vi "SaccadeAnalyser - Main.vi"(8 "error in (no error)":errorcluster, 11 "Data IN":T3={"Impulse Positions"=[{"Start"=5471, "End"=5813, "Impulse Plane"=enum."Yaw", "Impulse Direction +ve?"=FALSE, "Time offset"=0, "Amplitude offset"=0.0}, {"Start"=6974, "End"=7325, "Impulse Plane"=enum."Yaw", "Impulse Direction +ve?"=TRUE, "Time offset"=0, "Amplitude offset"=0.0}, {"Start"=7641, "End"=7980, "Impulse Plane"=enum."Yaw", "Impulse Direction +ve?"=FALSE, "Time offset"=0, "Amplitude offset"=0.0}, {"Start"=9060, "End"=9400, "Impulse Plane"=enum."Yaw", "Impulse Direction +ve?"=FALSE, "Time offset"=0, "Amplitude offset"=0.0}, {"Start"=9938, "End"=10282, "Impulse Plane"=enum."Yaw", "Impulse Direction +ve?"=FALSE, "Time offset"=0, "Amplitude offset"=0.0}, {"Start"=10800, "End"=11142, "Impulse Plane"=enum."Yaw", "Impulse Direction +ve?"=FALSE, "Time offset"=0, "Amplitude offset"=0.0}, {"Start"=11602, "End"=11942, "Impulse Plane"=enum."Yaw", "Impulse Direction +ve?"=TRUE, "Time offset"=0, "Amplitude offset"=0.0}, {"Start"=12449, "End"=12790, "Impulse Plane"=enum."Yaw", "Impulse Direction +ve?"=TRUE, "Time offset"=0, "Amplitude offset"=0.0}, {"Start"=13310, "End"=13653, "Impulse Plane"=enum."Yaw", "Impulse Direction +ve?"=TRUE, "Time offset"=0, "Amplitude offset"=0.0}, {"Start"=14191, "End"=14535, "Impulse Plane"=enum."Yaw", "Impulse Direction +ve?"=TRUE, "Time offset"=0, "Amplitude offset"=0.0}, {"Start"=15040, "End"=15380, "Impulse Plane"=enum."Yaw", "Impulse Direction +ve?"=FALSE, "Time offset"=0, "Amplitude offset"=0.0}, {"Start"=16780, "End"=17124, "Impulse Plane"=enum."Yaw", "Impulse Direction +ve?"=TRUE, "Time offset"=0, "Amplitude offset"=0.0}, {"Start"=17572, "End"=17913, "Impulse Plane"=enum."Yaw", "Impulse Direction +ve?"=FALSE, "Time offset"=0, "Amplitude offset"=0.0}, {"Start"=18369, "End"=18713, "Impulse Plane"=enum."Yaw", "Impulse Direction +ve?"=FALSE, "Time offset"=0, "Amplitude offset"=0.0}, {"Start"=19174, "End"=19519, "Impulse Plane"=enum."Yaw", "Impulse Direction +ve?"=FALSE, "Time offset"=0, "Amplitude offset"=0.0}, {"Start"=19928, "End"=20270, "Impulse Plane"=enum."Yaw", "Impulse Direction +ve?"=TRUE, "Time offset"=0, "Amplitude offset"=0.0}, {"Start"=20762, "End"=21121, "Impulse Plane"=enum."Yaw", "Impulse Direction +ve?"=FALSE, "Time offset"=0, "Amplitude offset"=0.0}, {"Start"=21554, "End"=21888, "Impulse Plane"=enum."Yaw", "Impulse Direction +ve?"=FALSE, "Time offset"=0, "Amplitude offset"=0.0}, {"Start"=22293, "End"=22639, "Impulse Plane"=enum."Yaw", "Impulse Direction +ve?"=TRUE, "Time offset"=0, "Amplitude offset"=0.0}, {"Start"=23109, "End"=23464, "Impulse Plane"=enum."Yaw", "Impulse Direction +ve?"=TRUE, "Time offset"=0, "Amplitude offset"=0.0}, {"Start"=23868, "End"=24215, "Impulse Plane"=enum."Yaw", "Impulse Direction +ve?"=TRUE, "Time offset"=0, "Amplitude offset"=0.0}, {"Start"=24643, "End"=24992, "Impulse Plane"=enum."Yaw", "Impulse Direction +ve?"=FALSE, "Time offset"=0, "Amplitude offset"=0.0}, {"Start"=25685, "End"=26023, "Impulse Plane"=enum."Yaw", "Impulse Direction +ve?"=FALSE, "Time offset"=0, "Amplitude offset"=0.0}, {"Start"=26431, "End"=26768, "Impulse Plane"=enum."Yaw", "Impulse Direction +ve?"=FALSE, "Time offset"=0, "Amplitude offset"=0.0}, {"Start"=27251, "End"=27595, "Impulse Plane"=enum."Yaw", "Impulse Direction +ve?"=FALSE, "Time offset"=0, "Amplitude offset"=0.0}, {"Start"=28832, "End"=29180, "Impulse Plane"=enum."Yaw", "Impulse Direction +ve?"=TRUE, "Time offset"=0, "Amplitude offset"=0.0}, {"Start"=31028, "End"=31383, "Impulse Plane"=enum."LARP", "Impulse Direction +ve?"=FALSE, "Time offset"=0, "Amplitude offset"=0.0}, {"Start"=32603, "End"=32936, "Impulse Plane"=enum."LARP", "Impulse Direction +ve?"=TRUE, "Time offset"=0, "Amplitude offset"=0.0}, {"Start"=33445, "End"=33779, "Impulse Plane"=enum."LARP", "Impulse Direction +ve?"=TRUE, "Time offset"=0, "Amplitude offset"=0.0}, {"Start"=34276, "End"=34629, "Impulse Plane"=enum."LARP", "Impulse Direction +ve?"=FALSE, "Time offset"=0, "Amplitude offset"=0.0}, {"Start"=35114, "End"=35460, "Impulse Plane"=enum."LARP", "Impulse Direction +ve?"=FALSE, "Time offset"=0, "Amplitude offset"=0.0}, {"Start"=35981, "End"=36324, "Impulse Plane"=enum."LARP", "Impulse Direction +ve?"=TRUE, "Time offset"=0, "Amplitude offset"=0.0}, {"Start"=36920, "End"=37249, "Impulse Plane"=enum."LARP", "Impulse Direction +ve?"=TRUE, "Time offset"=0, "Amplitude offset"=0.0}, {"Start"=37988, "End"=38322, "Impulse Plane"=enum."LARP", "Impulse Direction +ve?"=TRUE, "Time offset"=0, "Amplitude offset"=0.0}, {"Start"=38964, "End"=39324, "Impulse Plane"=enum."LARP", "Impulse Direction +ve?"=FALSE, "Time offset"=0, "Amplitude offset"=0.0}, {"Start"=39948, "End"=40284, "Impulse Plane"=enum."LARP", "Impulse Direction +ve?"=TRUE, "Time offset"=0, "Amplitude offset"=0.0}, {"Start"=40958, "End"=41293, "Impulse Plane"=enum."LARP", "Impulse Direction +ve?"=TRUE, "Time offset"=0, "Amplitude offset"=0.0}, {"Start"=41899, "End"=42229, "Impulse Plane"=enum."LARP", "Impulse Direction +ve?"=TRUE, "Time offset"=0, "Amplitude offset"=0.0}, {"Start"=42801, "End"=43154, "Impulse Plane"=enum."LARP", "Impulse Direction +ve?"=FALSE, "Time offset"=0, "Amplitude offset"=0.0}, {"Start"=43641, "End"=43980, "Impulse Plane"=enum."LARP", "Impulse Direction +ve?"=TRUE, "Time offset"=0, "Amplitude offset"=0.0}, {"Start"=44466, "End"=44821, "Impulse Plane"=enum."LARP", "Impulse Direction +ve?"=FALSE, "Time offset"=0, "Amplitude offset"=0.0}, {"Start"=45388, "End"=45722, "Impulse Plane"=enum."LARP", "Impulse Direction +ve?"=TRUE, "Time offset"=0, "Amplitude offset"=0.0}, {"Start"=46149, "End"=46510, "Impulse Plane"=enum."LARP", "Impulse Direction +ve?"=FALSE, "Time offset"=0, "Amplitude offset"=0.0}, {"Start"=47874, "End"=48206, "Impulse Plane"=enum."LARP", "Impulse Direction +ve?"=TRUE, "Time offset"=0, "Amplitude offset"=0.0}, {"Start"=50143, "End"=50479, "Impulse Plane"=enum."RALP", "Impulse Direction +ve?"=TRUE, "Time offset"=0, "Amplitude offset"=0.0}, {"Start"=50976, "End"=51310, "Impulse Plane"=enum."RALP", "Impulse Direction +ve?"=FALSE, "Time offset"=0, "Amplitude offset"=0.0}, {"Start"=51892, "End"=52226, "Impulse Plane"=enum."RALP", "Impulse Direction +ve?"=FALSE, "Time offset"=0, "Amplitude offset"=0.0}, {"Start"=52839, "End"=53171, "Impulse Plane"=enum."RALP", "Impulse Direction +ve?"=FALSE, "Time offset"=0, "Amplitude offset"=0.0}, {"Start"=53676, "End"=54012, "Impulse Plane"=enum."RALP", "Impulse Direction +ve?"=TRUE, "Time offset"=0, "Amplitude offset"=0.0}, {"Start"=54530, "End"=54877, "Impulse Plane"=enum."RALP", "Impulse Direction +ve?"=FALSE, "Time offset"=0, "Amplitude offset"=0.0}, {"Start"=55371, "End"=55711, "Impulse Plane"=enum."RALP", "Impulse Direction +ve?"=TRUE, "Time offset"=0, "Amplitude offset"=0.0}, {"Start"=56153, "End"=56482, "Impulse Plane"=enum."RALP", "Impulse Direction +ve?"=FALSE, "Time offset"=0, "Amplitude offset"=0.0}, {"Start"=57053, "End"=57390, "Impulse Plane"=enum."RALP", "Impulse Direction +ve?"=FALSE, "Time offset"=0, "Amplitude offset"=0.0}, {"Start"=57954, "End"=58292, "Impulse Plane"=enum."RALP", "Impulse Direction +ve?"=FALSE, "Time offset"=0, "Amplitude offset"=0.0}, {"Start"=58794, "End"=59130, "Impulse Plane"=enum."RALP", "Impulse Direction +ve?"=TRUE, "Time offset"=0, "Amplitude offset"=0.0}, {"Start"=59587, "End"=59931, "Impulse Plane"=enum."RALP", "Impulse Direction +ve?"=TRUE, "Time offset"=0, "Amplitude offset"=0.0}, {"Start"=60399, "End"=60744, "Impulse Plane"=enum."RALP", "Impulse Direction +ve?"=FALSE, "Time offset"=0, "Amplitude offset"=0.0}, {"Start"=61218, "End"=61559, "Impulse Plane"=enum."RALP", "Impulse Direction +ve?"=FALSE, "Time offset"=0, "Amplitude offset"=0.0}, {"Start"=62100, "End"=62442, "Impulse Plane"=enum."RALP", "Impulse Direction +ve?"=FALSE, "Time offset"=0, "Amplitude offset"=0.0}, {"Start"=62989, "End"=63322, "Impulse Plane"=enum."RALP", "Impulse Direction +ve?"=FALSE, "Time offset"=0, "Amplitude offset"=0.0}, {"Start"=63787, "End"=64136, "Impulse Plane"=enum."RALP", "Impulse Direction +ve?"=TRUE, "Time offset"=0, "Amplitude offset"=0.0}, {"Start"=64603, "End"=64953, "Impulse Plane"=enum."RALP", "Impulse Direction +ve?"=FALSE, "Time offset"=0, "Amplitude offset"=0.0}, {"Start"=65462, "End"=65795, "Impulse Plane"=enum."RALP", "Impulse Direction +ve?"=FALSE, "Time offset"=0, "Amplitude offset"=0.0}, {"Start"=66308, "End"=66645, "Impulse Plane"=enum."RALP", "Impulse Direction +ve?"=FALSE, "Time offset"=0, "Amplitude offset"=0.0}, {"Start"=67052, "End"=67402, "Impulse Plane"=enum."RALP", "Impulse Direction +ve?"=TRUE, "Time offset"=0, "Amplitude offset"=0.0}], "No. Imp"=15, "Parameter Time Series"=[{"time offset"=0.0, "Offset"=0.0, "Gain"=1.0, "inverse"=FALSE, "filter data"=FALSE, "dots"=FALSE, "interpolate"=FALSE, "List 1"=5, "Color Box"=6618880, "Boolean"=TRUE}, {"time offset"=0.0, "Offset"=0.0, "Gain"=1.0, "inverse"=FALSE, "filter data"=FALSE, "dots"=FALSE, "interpolate"=FALSE, "List 1"=6, "Color Box"=6618880, "Boolean"=FALSE}, {"time offset"=0.0, "Offset"=0.0, "Gain"=1.0, "inverse"=FALSE, "filter data"=FALSE, "dots"=FALSE, "interpolate"=FALSE, "List 1"=7, "Color Box"=6618880, "Boolean"=FALSE}, {"time offset"=0.0, "Offset"=0.0, "Gain"=1.0, "inverse"=FALSE, "filter data"=FALSE, "dots"=FALSE, "interpolate"=FALSE, "List 1"=13, "Color Box"=16777224, "Boolean"=TRUE}, {"time offset"=0.0, "Offset"=0.0, "Gain"=1.0, "inverse"=FALSE, "filter data"=FALSE, "dots"=FALSE, "interpolate"=FALSE, "List 1"=14, "Color Box"=16777224, "Boolean"=FALSE}, {"time offset"=0.0, "Offset"=0.0, "Gain"=1.0, "inverse"=FALSE, "filter data"=FALSE, "dots"=FALSE, "interpolate"=FALSE, "List 1"=15, "Color Box"=16777224, "Boolean"=FALSE}], "Parameter Impuls Series"=[{"Color"=6618880, "Visible"=TRUE, "Channel"=1, "Invert"=FALSE, "Desaccade"=FALSE, "Offset"=0.0, "Gain"=1.0}, {"Color"=6618880, "Visible"=FALSE, "Channel"=6, "Invert"=FALSE, "Desaccade"=FALSE, "Offset"=0.0, "Gain"=1.0}, {"Color"=6618880, "Visible"=FALSE, "Channel"=7, "Invert"=FALSE, "Desaccade"=FALSE, "Offset"=0.0, "Gain"=1.0}, {"Color"=16777224, "Visible"=TRUE, "Channel"=13, "Invert"=FALSE, "Desaccade"=FALSE, "Offset"=0.0, "Gain"=1.0}, {"Color"=16777224, "Visible"=FALSE, "Channel"=14, "Invert"=FALSE, "Desaccade"=FALSE, "Offset"=0.0, "Gain"=1.0}, {"Color"=16777224, "Visible"=FALSE, "Channel"=15, "Invert"=FALSE, "Desaccade"=FALSE, "Offset"=0.0, "Gain"=1.0}], "Experiment Parameters"={"Freq"=0.0, "Vel"=0, "Acc"=0, "Stimulus"="Head Impulse"}, "Autosort File"=refnum, "Data File"={"Data Channels"=array34x71049[2415666 elements], "Sample Rate"=500, "Channel List"=["Hz Position-in-Head", "Hz Velocity-in-Head", "Hy Position-in-Head", "Hy Velocity-in-Head", "Hx Position-in-Head", "Hx Velocity-in-Head", "Hl Velocity-in-Head", "Hr Velocity-in-Head", "Lx Position-in-Head", "Ly Position-in-Head", "Lz Position-in-Head", "Lx Velocity-in-Head", "Ly Velocity-in-Head", "Lz Velocity-in-Head", "Ll Velocity-in-Head", "Lr Velocity-in-Head", "Rx Position-in-Head", "Ry Position-in-Head", "Rz Position-in-Head", "Rx Velocity-in-Head", "Ry Velocity-in-Head", "Rz Velocity-in-Head", "Rl Velocity-in-Head", "Rr Velocity-in-Head", "Target on/off", "aux input 1", "aux input 2", " ", "", "", "", "Target Hor", "Target Ver", ""]}, "Experiment data path"=path "C:/Users/w.figtree/Desktop/Coils Data/3", "Image data path"=path "/Macintosh HD/Users/patrick/Studium/Diploma Thesis/Data Analysis", "LVS data path"=path "/Macintosh HD/Users/patrick/Studium/Diploma Thesis/Data Analysis", "Raw copy path"=path "/Macintosh HD/Users/patrick/Studium/Diploma Thesis/Data Analysis", "filename"="passive_lvs.lvs", "desaccading parameters"={"Tolerance"=3, "Acc Range"=7000.0, "Sample Rate"=500, "Impulse Plane 2"=enum."Yaw", "Impulse dir"=FALSE}, "Experiment Parameters 2"={"Subject"="SE Trial Short Term", "Strain"="", "Rotation plane"="", "Experimenter"=" ", "Trial"=0.0, "Time"=0.0}, "Excel"={"Excel._Application"=refnum, "Use Excel"=TRUE, "Worksheet SINE"=refnum, "Row SINE"=0, "Worksheet TRANS"=refnum, "Row TRANS"=0}, "Session Config File"=refnum, "Autosort Parameter Set"=4, "EMA Version"="EMA 2016a", "desacc "={"Threshold 1 [Acc]"=7000.0, "Threshold 2 [% of TH1]"=60, "tolerance"=3, "Search WD "=0.1, " always use TH2"=FALSE, "Range"=3.0, "Max time"=120.0, "Min time"=20.0, "Velocity Threshold"=150}, "Cycle Nr for Saccades"={"POS"=0, "NEG"=0}, "calibration name"="u_calibration_1_p00001s001_calib.mat", "Excel"=refnum} {"Parameter Time Series"."time offset" format="%.3f"; "Parameter Time Series"."Gain" format="%.1f"; "Parameter Time Series"."Offset" format="%.1f"; "Parameter Time Series"."List 1" items=["Motor-Pos", "Motor-Vel", "Lx Position-in-Head", "Ly Position-in-Head", "Lz Position-in-Head", "Lx Velocity-in-Head", "Ly Velocity-in-Head", "Lz Velocity-in-Head", "Ll Velocity-in-Head", "Lr Velocity-in-Head", "Lx Accel-in-Head", "Ly Accel-in-Head", "Lz Accel-in-Head", "Rx Position-in-Head", "Ry Position-in-Head", "Rz Position-in-Head", "Rx Velocity-in-Head", "Ry Velocity-in-Head", "Rz Velocity-in-Head", "Rl Velocity-in-Head", "Rr Velocity-in-Head", "Rx Accel-in-Head", "Ry Accel-in-Head", "Rz Accel-in-Head", "Global Trigger", "", "", ""]; "Parameter Impuls Series"."Gain" format="%.1f"; "Parameter Impuls Series"."Offset" format="%.1f"}) -> (0 "error out":errorcluster, 3 "Data OUT":T3={"Impulse Positions"=[{"Start"=5471, "End"=5813, "Impulse Plane"=enum."Yaw", "Impulse Direction +ve?"=FALSE, "Time offset"=0, "Amplitude offset"=0.0}, {"Start"=6974, "End"=7325, "Impulse Plane"=enum."Yaw", "Impulse Direction +ve?"=TRUE, "Time offset"=0, "Amplitude offset"=0.0}, {"Start"=7641, "End"=7980, "Impulse Plane"=enum."Yaw", "Impulse Direction +ve?"=FALSE, "Time offset"=0, "Amplitude offset"=0.0}, {"Start"=9060, "End"=9400, "Impulse Plane"=enum."Yaw", "Impulse Direction +ve?"=FALSE, "Time offset"=0, "Amplitude offset"=0.0}, {"Start"=9938, "End"=10282, "Impulse Plane"=enum."Yaw", "Impulse Direction +ve?"=FALSE, "Time offset"=0, "Amplitude offset"=0.0}, {"Start"=10800, "End"=11142, "Impulse Plane"=enum."Yaw", "Impulse Direction +ve?"=FALSE, "Time offset"=0, "Amplitude offset"=0.0}, {"Start"=11602, "End"=11942, "Impulse Plane"=enum."Yaw", "Impulse Direction +ve?"=TRUE, "Time offset"=0, "Amplitude offset"=0.0}, {"Start"=12449, "End"=12790, "Impulse Plane"=enum."Yaw", "Impulse Direction +ve?"=TRUE, "Time offset"=0, "Amplitude offset"=0.0}, {"Start"=13310, "End"=13653, "Impulse Plane"=enum."Yaw", "Impulse Direction +ve?"=TRUE, "Time offset"=0, "Amplitude offset"=0.0}, {"Start"=14191, "End"=14535, "Impulse Plane"=enum."Yaw", "Impulse Direction +ve?"=TRUE, "Time offset"=0, "Amplitude offset"=0.0}, {"Start"=15040, "End"=15380, "Impulse Plane"=enum."Yaw", "Impulse Direction +ve?"=FALSE, "Time offset"=0, "Amplitude offset"=0.0}, {"Start"=16780, "End"=17124, "Impulse Plane"=enum."Yaw", "Impulse Direction +ve?"=TRUE, "Time offset"=0, "Amplitude offset"=0.0}, {"Start"=17572, "End"=17913, "Impulse Plane"=enum."Yaw", "Impulse Direction +ve?"=FALSE, "Time offset"=0, "Amplitude offset"=0.0}, {"Start"=18369, "End"=18713, "Impulse Plane"=enum."Yaw", "Impulse Direction +ve?"=FALSE, "Time offset"=0, "Amplitude offset"=0.0}, {"Start"=19174, "End"=19519, "Impulse Plane"=enum."Yaw", "Impulse Direction +ve?"=FALSE, "Time offset"=0, "Amplitude offset"=0.0}, {"Start"=19928, "End"=20270, "Impulse Plane"=enum."Yaw", "Impulse Direction +ve?"=TRUE, "Time offset"=0, "Amplitude offset"=0.0}, {"Start"=20762, "End"=21121, "Impulse Plane"=enum."Yaw", "Impulse Direction +ve?"=FALSE, "Time offset"=0, "Amplitude offset"=0.0}, {"Start"=21554, "End"=21888, "Impulse Plane"=enum."Yaw", "Impulse Direction +ve?"=FALSE, "Time offset"=0, "Amplitude offset"=0.0}, {"Start"=22293, "End"=22639, "Impulse Plane"=enum."Yaw", "Impulse Direction +ve?"=TRUE, "Time offset"=0, "Amplitude offset"=0.0}, {"Start"=23109, "End"=23464, "Impulse Plane"=enum."Yaw", "Impulse Direction +ve?"=TRUE, "Time offset"=0, "Amplitude offset"=0.0}, {"Start"=23868, "End"=24215, "Impulse Plane"=enum."Yaw", "Impulse Direction +ve?"=TRUE, "Time offset"=0, "Amplitude offset"=0.0}, {"Start"=24643, "End"=24992, "Impulse Plane"=enum."Yaw", "Impulse Direction +ve?"=FALSE, "Time offset"=0, "Amplitude offset"=0.0}, {"Start"=25685, "End"=26023, "Impulse Plane"=enum."Yaw", "Impulse Direction +ve?"=FALSE, "Time offset"=0, "Amplitude offset"=0.0}, {"Start"=26431, "End"=26768, "Impulse Plane"=enum."Yaw", "Impulse Direction +ve?"=FALSE, "Time offset"=0, "Amplitude offset"=0.0}, {"Start"=27251, "End"=27595, "Impulse Plane"=enum."Yaw", "Impulse Direction +ve?"=FALSE, "Time offset"=0, "Amplitude offset"=0.0}, {"Start"=28832, "End"=29180, "Impulse Plane"=enum."Yaw", "Impulse Direction +ve?"=TRUE, "Time offset"=0, "Amplitude offset"=0.0}, {"Start"=31028, "End"=31383, "Impulse Plane"=enum."LARP", "Impulse Direction +ve?"=FALSE, "Time offset"=0, "Amplitude offset"=0.0}, {"Start"=32603, "End"=32936, "Impulse Plane"=enum."LARP", "Impulse Direction +ve?"=TRUE, "Time offset"=0, "Amplitude offset"=0.0}, {"Start"=33445, "End"=33779, "Impulse Plane"=enum."LARP", "Impulse Direction +ve?"=TRUE, "Time offset"=0, "Amplitude offset"=0.0}, {"Start"=34276, "End"=34629, "Impulse Plane"=enum."LARP", "Impulse Direction +ve?"=FALSE, "Time offset"=0, "Amplitude offset"=0.0}, {"Start"=35114, "End"=35460, "Impulse Plane"=enum."LARP", "Impulse Direction +ve?"=FALSE, "Time offset"=0, "Amplitude offset"=0.0}, {"Start"=35981, "End"=36324, "Impulse Plane"=enum."LARP", "Impulse Direction +ve?"=TRUE, "Time offset"=0, "Amplitude offset"=0.0}, {"Start"=36920, "End"=37249, "Impulse Plane"=enum."LARP", "Impulse Direction +ve?"=TRUE, "Time offset"=0, "Amplitude offset"=0.0}, {"Start"=37988, "End"=38322, "Impulse Plane"=enum."LARP", "Impulse Direction +ve?"=TRUE, "Time offset"=0, "Amplitude offset"=0.0}, {"Start"=38964, "End"=39324, "Impulse Plane"=enum."LARP", "Impulse Direction +ve?"=FALSE, "Time offset"=0, "Amplitude offset"=0.0}, {"Start"=39948, "End"=40284, "Impulse Plane"=enum."LARP", "Impulse Direction +ve?"=TRUE, "Time offset"=0, "Amplitude offset"=0.0}, {"Start"=40958, "End"=41293, "Impulse Plane"=enum."LARP", "Impulse Direction +ve?"=TRUE, "Time offset"=0, "Amplitude offset"=0.0}, {"Start"=41899, "End"=42229, "Impulse Plane"=enum."LARP", "Impulse Direction +ve?"=TRUE, "Time offset"=0, "Amplitude offset"=0.0}, {"Start"=42801, "End"=43154, "Impulse Plane"=enum."LARP", "Impulse Direction +ve?"=FALSE, "Time offset"=0, "Amplitude offset"=0.0}, {"Start"=43641, "End"=43980, "Impulse Plane"=enum."LARP", "Impulse Direction +ve?"=TRUE, "Time offset"=0, "Amplitude offset"=0.0}, {"Start"=44466, "End"=44821, "Impulse Plane"=enum."LARP", "Impulse Direction +ve?"=FALSE, "Time offset"=0, "Amplitude offset"=0.0}, {"Start"=45388, "End"=45722, "Impulse Plane"=enum."LARP", "Impulse Direction +ve?"=TRUE, "Time offset"=0, "Amplitude offset"=0.0}, {"Start"=46149, "End"=46510, "Impulse Plane"=enum."LARP", "Impulse Direction +ve?"=FALSE, "Time offset"=0, "Amplitude offset"=0.0}, {"Start"=47874, "End"=48206, "Impulse Plane"=enum."LARP", "Impulse Direction +ve?"=TRUE, "Time offset"=0, "Amplitude offset"=0.0}, {"Start"=50143, "End"=50479, "Impulse Plane"=enum."RALP", "Impulse Direction +ve?"=TRUE, "Time offset"=0, "Amplitude offset"=0.0}, {"Start"=50976, "End"=51310, "Impulse Plane"=enum."RALP", "Impulse Direction +ve?"=FALSE, "Time offset"=0, "Amplitude offset"=0.0}, {"Start"=51892, "End"=52226, "Impulse Plane"=enum."RALP", "Impulse Direction +ve?"=FALSE, "Time offset"=0, "Amplitude offset"=0.0}, {"Start"=52839, "End"=53171, "Impulse Plane"=enum."RALP", "Impulse Direction +ve?"=FALSE, "Time offset"=0, "Amplitude offset"=0.0}, {"Start"=53676, "End"=54012, "Impulse Plane"=enum."RALP", "Impulse Direction +ve?"=TRUE, "Time offset"=0, "Amplitude offset"=0.0}, {"Start"=54530, "End"=54877, "Impulse Plane"=enum."RALP", "Impulse Direction +ve?"=FALSE, "Time offset"=0, "Amplitude offset"=0.0}, {"Start"=55371, "End"=55711, "Impulse Plane"=enum."RALP", "Impulse Direction +ve?"=TRUE, "Time offset"=0, "Amplitude offset"=0.0}, {"Start" (continued)
  T8 = typedef "Saccade Analyser Saccade Data.ctl" = cluster{"Impulse":i32, "Sequence #":dbl, "Start (idx)":dbl, "End (idx)":dbl, "Peak (idx)":dbl, "Onset (ms)":dbl, "Duration (ms)":dbl, "Vel (°/s)":dbl, "Amplitude (°)":dbl, "Gain":dbl, "Included?":bool}
  T9 = typedef "Saccade Analyser Summary Data.ctl" = cluster{"Num Impulses":dbl, "Num Saccades":dbl, "Onset (ms)":dbl, "Onset SD (ms)":dbl, "Duration (ms)":dbl, "Duration SD (ms)":dbl, "Vel (°/s)":dbl, "Vel SD (°/s)":dbl, "Amplitude (°)":dbl, "Amplitude SD (°)":dbl, "Gain":dbl, "Gain SD":dbl}
  T10 = typedef "Saccade Analyser States.ctl" = enum16{"Initialise", "Quit", "DO - Analysis", "DO - Summary Analysis", "Load Channel Data", "Find Impulses", "Find Saccades", "Sequence Saccades", "Calc Saccade Summary Stats", "Calc Saccade Group Stats", "DO - Draw", "Clear Plot", "Plot Selected Saccade", "Plot Selected Saccade Siblings", "Plot Impulse Data", "Plot Saccade Data", "Fill Saccade MCLB", "Fill Summary Stats", "Give MCLB Focus", "Halt Panel Updates", "Resume Panel Updates", "Disable Controls", "Enable Controls", "Toggle Saccade", "DO - Export Summary", "Export - Open Summary", "Export - Summary", "DO - Export Saccades", "Export - Open Saccades", "Export - Saccades", "DO - Export Group", "Export - Open Group", "Export - Group", "Do - Export All"}
  T11 = typedef "LVPoint32TypeDef.ctl" = cluster{"Horizontal":i32, "Vertical":i32}
  T12 = typedef "LVRowAndColumnTypeDef.ctl" = cluster{"Row":i32, "Column":i32}
  T13 = typedef "eventvkey.ctl" = enum16{"ASCII", "Enter", "Return", "Shift", "Ctrl", "Alt", "Cmd", "Opt", "Caps", "NumLock", "Clear", "Break", "Up", "Down", "Left", "Right", "Insert", "Delete", "Home", "End", "PageUp", "PageDown", "Escape", "Help", "Pause", "ScrollLock", "F1", "F2", "F3", "F4", "F5", "F6", "F7", "F8", "F9", "F10", "F11", "F12", "F13", "F14", "F15", "F16", "F17", "F18", "F19", "F20", "F21", "F22", "F23", "F24", "Play", "VolumeUp", "VolumeDown", "Mute", "Two Byte Char"}
  T14 = enum16{"Other", "Yaw", "Pitch", "Roll", "LARP", "RALP"}
  T15 = typedef "Saccade Analyser Impulse Data.ctl" = cluster{"Stimulus Data":dbl[], "Response Data":dbl[], "Response Pos Data":dbl[], "Peak (idx)":i32, "Onset (idx)":i32}
  T16 = cluster{"Channels":string[], "Impulse Plane":enum16{"Other", "Yaw", "Pitch", "Roll", "LARP", "RALP"}, "Impulse Direction +ve?":bool}
  T17 = cluster{"Plot.Anti-aliased":bool, "Plot.Bar Plot Style":u8, "Plot.Digital Line Style":u8, "Plot.Digital Transition Location":u8, "Plot.Digital Transition Type":u8, "Plot.Fill To":i16, "Plot.Fill/Point Color":u32, "Plot.Label Format":u8, "Plot.Line Style":u8, "Plot.Line Width":u8, "Plot.Plot Color":u32, "Plot.Plot Interpolation":u8, "Plot.Plot Name":string, "Plot.Point Style":u8, "Plot.Visible":bool}
  T18 = enum8{"Enabled", "Disabled", "Disabled and Grayed Out"}
  T19 = cluster{"Data Channels":dbl[][], "Sample Rate":i32, "Channel List":string[]}
  T20 = cluster{"Start":i32, "End":i32, "Impulse Plane":enum16{"Other", "Yaw", "Pitch", "Roll", "LARP", "RALP"}, "Impulse Direction +ve?":bool, "Time offset":i32, "Amplitude offset":dbl}[]
  T21 = cluster{dbl, "sac_AccMin":dbl, "sac_AccMult":dbl, "sac_BiphasicCond":dbl}
  T22 = cluster{"[0]":dbl, "[1]":dbl, "[2]":dbl, "[3]":dbl, "[4]":dbl, "[5]":dbl, "[6]":dbl, "[7]":dbl, "[8]":dbl, "[9]":dbl, "[10]":dbl, "[11]":dbl}
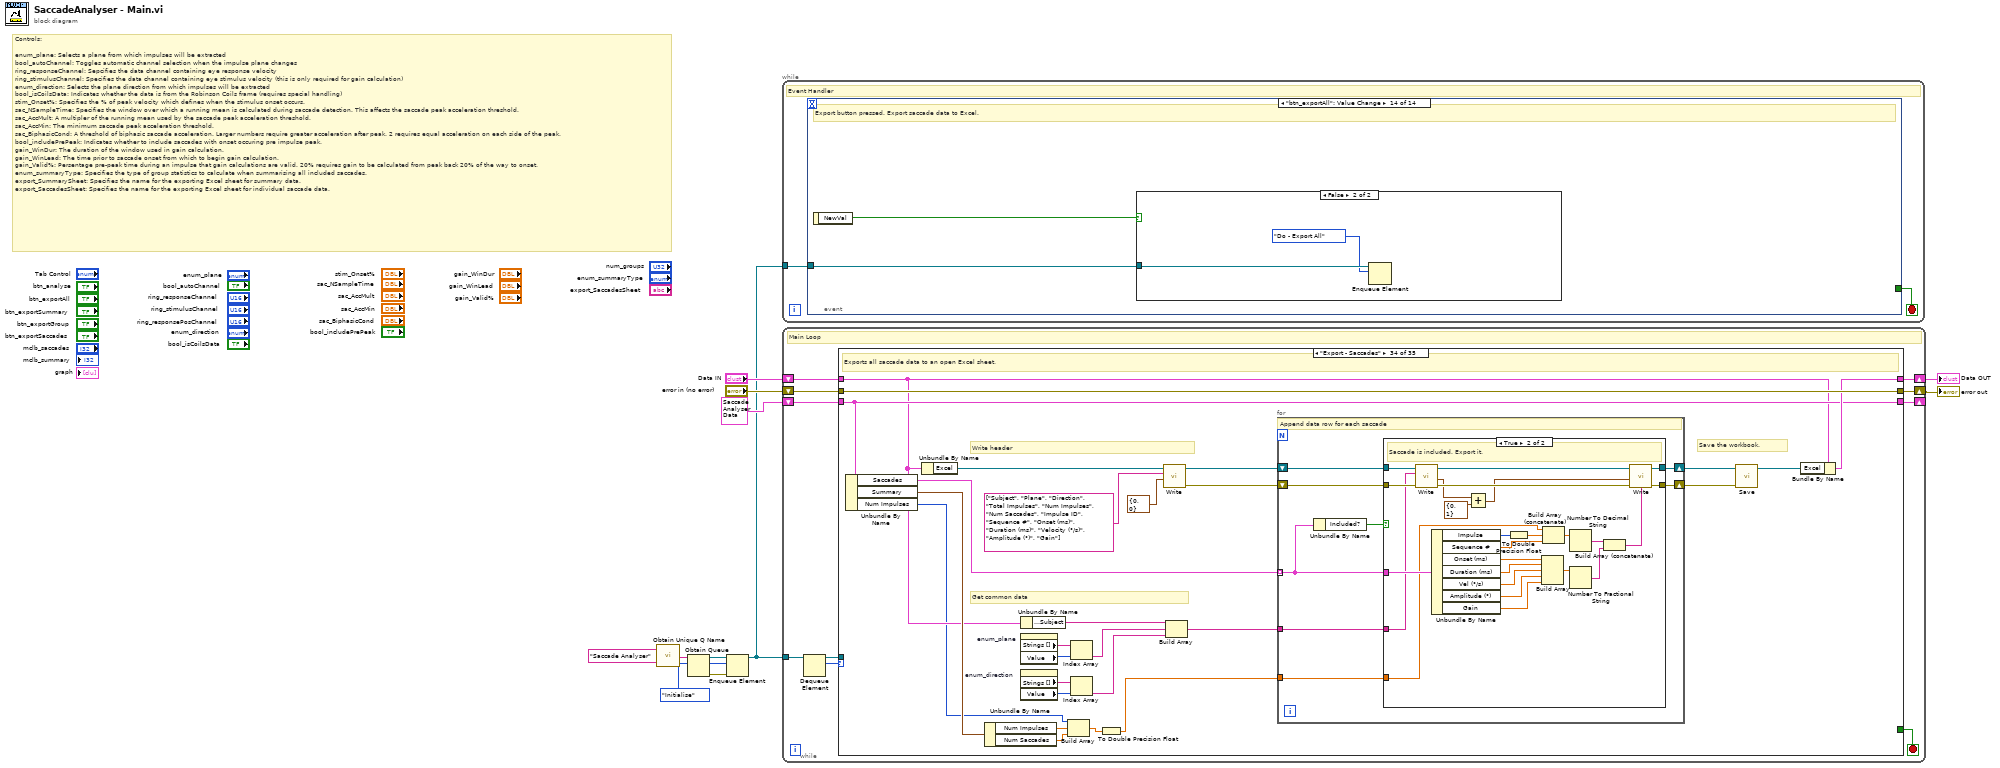
[diagram p0: block diagram]
diagram:
  w1 = Saccade_Analyser_States."Initialise" ("Saccade Analyser States")
  # "Controls:\n\nenum_plane: Selects a plane from which impulses will be extracted\nbool_autoChannel: Toggles automatic channel selection when the impulse plane changes\nring_responseChannel: Sepcifies the data channel containing eye response velocity\nring_stimulusChannel: Specifies the data channel containing eye stimulus velocity (this is only required for gain calculation)\nenum_direction: Selects the plane direction from which impulses will be extracted\nbool_isCoilsData: Indicates whether the data is from the Robinson Coils frame (requires special handling)\nstim_Onset%: Specifies the % of peak velocity which defines when the stimulus onset occurs.\nsac_NSampleTime: Specifies the window over which a running mean is calculated during saccade detection. This affects the saccade peak acceleration threshold.\nsac_AccMult: A multipler of the running mean used by the saccade peak acceleration threshold.\nsac_AccMin: The minimum saccade peak acceleration threshold.\nsac_BiphasicCond: A threshold of biphasic saccade acceleration. Larger numbers require greater acceleration after peak. 2 requires equal acceleration on each side of the peak.\nbool_includePrePeak: Indicates whether to include saccades with onset occuring pre impulse peak.\ngain_WinDur: The duration of the window used in gain calculation.\ngain_WinLead: The time prior to saccade onset from which to begin gain calculation.\ngain_Valid%: Persentage pre-peak time during an impulse that gain calculations are valid. 20% requires gain to be calculated from peak back 20% of the way to onset.\nenum_summaryType: Specifies the type of group statistics to calculate when summarising all included saccades.\nexport_SummarySheet: Specifies the name for the exporting Excel sheet for summary data.\nexport_SaccadesSheet: Specifies the name for the exporting Excel sheet for individual saccade data."
  n1 = call <userlib>:"Obtain Unique Q Name.vi"("Queue"="Saccade Analyser") -> ("Q Name"=w11:string)  [unwired: 4 in]
  n2 = Obtain Queue(name (unnamed)=w11, element data type=w1) -> (queue out=w4:refnum<queue>, error out=w3:errorcluster)  [unwired: 3 in, 1 out]
  n3 = Enqueue Element(queue=w4, element=w1, error in (no error)=w3) -> (queue out=w2:refnum<queue>)  [unwired: 1 in, 2 out]
  n4 = while {
    tunnel: w2 -> [w12]
    stop <- w13 stop-if-true
    # "Event Handler"
    n5 = event shown="[13] \"btn_exportAll\": Value Change" {
      selector: _ -> [_ _ _ _ _ _ _ _ _ _ _ _ _ _]
      dyn-events: _ -> [_ _ _ _ _ _ _ _ _ _ _ _ _ _]
      timeout: _ -> [_ _ _ _ _ _ _ _ _ _ _ _ _ _]
      tunnel: [_ TRUE _ _ _ _ _ _ _ _ _ _ _ _] -> w13
      tunnel: w12 -> [_ w15 w18 _ w50 w58 w59 w92 w101 w103 w105 w109 w113 w117]
      event Timeout {
        # "Never occurs."
        n6 = event-data() -> ()  [unwired: 1 in, 3 out]
      }
      event Panel Close? {
        # "User has requested the window close. End VI."
        n7 = event-data() -> ()  [unwired: 1 in, 4 out]
        n8 = Enqueue Element(queue=w15, element=Saccade_Analyser_States."Quit") -> ()  [unwired: 2 in, 3 out]
        n9 = call <userlib>:"Is Development Environment.vi"() -> ("exe?"=w16:bool)  [unwired: 5 in]
        n10 = event-data("Discard?"=w16) -> ()  [unwired: 1 in, 1 out]
      }
      event "btn_analyse": Value Change {
        # "Analysis button pressed. Do analysis."
        n11 = event-data() -> ("NewVal"=w19:bool)  [unwired: 1 in]
        n12 = case shown="False" w19 {
          tunnel: w18 -> [w20 _]
          frame False {
            n13 = Enqueue Element(queue=w20, element=Saccade_Analyser_States."DO - Analysis") -> ()  [unwired: 2 in, 3 out]
          }
          frame True {
          }
        }
      }
      event "mclb_saccades": Shortcut Menu Activation? {
        # "Is the clicked row in the bounds of the control and both populated and not the header."
        # "User has right clicked the MCLB. Create an Include/Exclude option."
        n14 = event-data() -> ("CtlRef"=w38:refnum<vi>, "Coords"=w37:T11, "MenuRef"=w35:refnum<k9>)  [unwired: 1 in]
        n15 = invoke class="MCListbox (strict)" method="Point To Row Column"(reference=w38, "Point"=w37) -> (reference out=w40:refnum<vi>, error out=w39:errorcluster, "InBounds"=w26:bool, "CellPosition"=w36:T12)  [unwired: 5 in, 3 out]
        n16 = Delete Menu Items(9:w35) -> (0:w42:errorcluster, 3:w41:refnum<k9>)  [unwired: 3 in]
        n17 = property class="MCListbox (strict)" props=["DisabledItems", "ItemNames"](reference=w40, error in=w39) -> (reference out=w23:refnum<vi>, error out=w22:errorcluster, "ItemNames"=w34:string[][])  [unwired: 1 out]
        n18 = Array Size(array=w34) -> (size(s)=w33:i32[])
        n19 = Unbundle By Name(w36) -> ("Row"=w32:i32)
        n20 = Index Array(array=w33) -> (element=w30:i32)  [unwired: 1 in]
        n21 = Decrement(x=w30) -> (x-1=w29:i32)
        n22 = In Range and Coerce(upper limit=w29, x=w32, lower limit=0) -> (coerced(x)=w28:i32, In Range?=w27:bool)
        n23 = And(x=w27, y=w26) -> (x .and. y?=w25:bool)
        n24 = case shown="True" w25 {
          tunnel: w42 -> [_ w49]
          tunnel: w41 -> [_ w48]
          tunnel: w28 -> [_ w44]
          tunnel: w23 -> [_ w46]
          tunnel: w22 -> [_ w45]
          frame False {
          }
          frame True {
            # "Select clicked row."
            n25 = property class="MCListbox (strict)"(reference=w46, error in=w45, "Value"=w44) -> ()  [unwired: 2 out]
            n26 = Build Array("Toggle Inclusion") -> (w47:string[])
            n27 = Insert Menu Items(6:w49, 8:w47, 9:w48) -> ()  [unwired: 3 in, 3 out]
          }
        }
        n28 = event-data("Discard?"=FALSE) -> ()  [unwired: 1 in, 1 out]
      }
      event "mclb_saccades": Shortcut Menu Selection (User) {
        # "The user has selected a shortcut menu item."
        n29 = event-data() -> ("ItemTag"=w51:string)  [unwired: 1 in, 2 out]
        n30 = case shown="\"Toggle Inclusion\"" w51 {
          tunnel: w50 -> [_ w54]
          frame Default {
            # "Unhandled menu selection."
            n31 = One Button Dialog(message="Unhandled right click menu selection.") -> ()  [unwired: 1 in, 1 out]
          }
          frame "Toggle Inclusion" {
            w53 = T10[] [enum."Toggle Saccade", enum."DO - Summary Analysis"] items=["Initialise", "Quit", "DO - Analysis", "DO - Summary Analysis", "Load Channel Data", "Find Impulses", "Find Saccades", "Sequence Saccades", "Calc Saccade Summary Stats", "Calc Saccade Group Stats", "DO - Draw", "Clear Plot", "Plot Selected Saccade", "Plot Selected Saccade Siblings", "Plot Impulse Data", "Plot Saccade Data", "Fill Saccade MCLB", "Fill Summary Stats", "Give MCLB Focus", "Halt Panel Updates", "Resume Panel Updates", "Disable Controls", "Enable Controls", "Toggle Saccade", "DO - Export Summary", "Export - Open Summary", "Export - Summary", "DO - Export Saccades", "Export - Open Saccades", "Export - Saccades", "DO - Export Group", "Export - Open Group", "Export - Group", "Do - Export All"] ("element")
            # "User has opted to toggle the saccade inclusion status."
            n32 = for {
              tunnel: w54 -> [w56]
              tunnel: w53 -> [w55] mode=indexing
              n33 = Enqueue Element(queue=w56, element=w55) -> ()  [unwired: 2 in, 3 out]
            }
          }
        }
      }
      event "mclb_saccades": Value Change {
        # "A new saccade has been selected. Redraw."
        n34 = event-data() -> ()  [unwired: 1 in, 6 out]
        n35 = Enqueue Element(queue=w58, element=Saccade_Analyser_States."DO - Draw") -> ()  [unwired: 2 in, 3 out]
      }
      event Key Down {
        # "User has pressed a key. Handle as appropriate."
        n36 = event-data() -> ("Char"=w61:i16, "VKey"=w62:T13, "ScanCode"=w60:i16)  [unwired: 1 in]
        n37 = case shown="\"Right\"" w62 {
          tunnel: w61 -> [_ _ _ _ _ _]
          tunnel: w60 -> [_ _ w67 _ _ _]
          tunnel: w59 -> [_ w63 _ _ _ w86]
          frame Default {
            # "Unhandled key press."
          }
          frame "Clear", "Delete", "Escape" {
            w64 = T10[] [enum."Toggle Saccade", enum."DO - Summary Analysis"] items=["Initialise", "Quit", "DO - Analysis", "DO - Summary Analysis", "Load Channel Data", "Find Impulses", "Find Saccades", "Sequence Saccades", "Calc Saccade Summary Stats", "Calc Saccade Group Stats", "DO - Draw", "Clear Plot", "Plot Selected Saccade", "Plot Selected Saccade Siblings", "Plot Impulse Data", "Plot Saccade Data", "Fill Saccade MCLB", "Fill Summary Stats", "Give MCLB Focus", "Halt Panel Updates", "Resume Panel Updates", "Disable Controls", "Enable Controls", "Toggle Saccade", "DO - Export Summary", "Export - Open Summary", "Export - Summary", "DO - Export Saccades", "Export - Open Saccades", "Export - Saccades", "DO - Export Group", "Export - Open Group", "Export - Group", "Do - Export All"] ("element")
            # "Include/Exclude selected saccade. (\"Clear\" = \"5\" on the numpad)"
            n38 = for {
              tunnel: w63 -> [w66]
              tunnel: w64 -> [w65] mode=indexing
              n39 = Enqueue Element(queue=w66, element=w65) -> ()  [unwired: 2 in, 3 out]
            }
          }
          frame "ASCII" {
            n40 = case shown="74" w67 {
              frame Default {
              }
              frame 78 {
                # "Plus Key"
                n41 = property on="enum_direction" class="Enum (strict)"("Val(Sgnl)"=enum16{"Positive", "Negative"}."Positive" ("Value (Signaling)")) -> ()  [unwired: 2 in, 2 out]
              }
              frame 74 {
                # "Minus Key"
                n42 = property on="enum_direction" class="Enum (strict)"("Val(Sgnl)"=enum16{"Positive", "Negative"}."Negative" ("Value (Signaling)")) -> ()  [unwired: 2 in, 2 out]
              }
            }
          }
          frame "Left" {
            n43 = property on="enum_plane" class="Enum (strict)"() -> ("Strings []"=w75:string[], "Value"=w76:T14)  [unwired: 2 in, 2 out]
            n44 = Array Size(array=w75) -> (size(s)=w74:i32)
            n45 = Decrement(x=w76) -> (x-1=w71:T14)
            n46 = Decrement(x=w74) -> (x-1=w72:i32)
            n47 = Less Than 0?(x=w71) -> (x < 0?=w73:bool)
            n48 = Select(t=w72, s=w73, f=w71) -> (s? t:f=w70:i32)
            n49 = property on="enum_plane" class="Enum (strict)"("Val(Sgnl)"=w70) -> ()  [unwired: 2 in, 2 out]
          }
          frame "Right" {
            n50 = property on="enum_plane" class="Enum (strict)"() -> ("Strings []"=w83:string[], "Value"=w84:T14)  [unwired: 2 in, 2 out]
            n51 = Array Size(array=w83) -> (size(s)=w82:i32)
            n52 = Increment(x=w84) -> (x+1=w80:T14)
            n53 = Decrement(x=w82) -> (x-1=w79:i32)
            n54 = Greater?(x=w80, y=w79) -> (0:w78:bool)
            n55 = Select(t=0, s=w78, f=w80) -> (s? t:f=w81:i32)
            n56 = property on="enum_plane" class="Enum (strict)"("Val(Sgnl)"=w81) -> ()  [unwired: 2 in, 2 out]
          }
          frame "Enter" {
            # "Enter pressed -> Export"
            n57 = disable-structure shown="Enabled" {
              disable-tunnel: [w87 w88] -> w85
              frame Disabled {
                w87 = T10[] [enum."DO - Export Summary", enum."DO - Export Saccades"] items=["Initialise", "Quit", "DO - Analysis", "DO - Summary Analysis", "Load Channel Data", "Find Impulses", "Find Saccades", "Sequence Saccades", "Calc Saccade Summary Stats", "Calc Saccade Group Stats", "DO - Draw", "Clear Plot", "Plot Selected Saccade", "Plot Selected Saccade Siblings", "Plot Impulse Data", "Plot Saccade Data", "Fill Saccade MCLB", "Fill Summary Stats", "Give MCLB Focus", "Halt Panel Updates", "Resume Panel Updates", "Disable Controls", "Enable Controls", "Toggle Saccade", "DO - Export Summary", "Export - Open Summary", "Export - Summary", "DO - Export Saccades", "Export - Open Saccades", "Export - Saccades", "DO - Export Group", "Export - Open Group", "Export - Group", "Do - Export All"] ("element")
              }
              frame Enabled {
                w88 = T10[] [enum."DO - Export Saccades"] items=["Initialise", "Quit", "DO - Analysis", "DO - Summary Analysis", "Load Channel Data", "Find Impulses", "Find Saccades", "Sequence Saccades", "Calc Saccade Summary Stats", "Calc Saccade Group Stats", "DO - Draw", "Clear Plot", "Plot Selected Saccade", "Plot Selected Saccade Siblings", "Plot Impulse Data", "Plot Saccade Data", "Fill Saccade MCLB", "Fill Summary Stats", "Give MCLB Focus", "Halt Panel Updates", "Resume Panel Updates", "Disable Controls", "Enable Controls", "Toggle Saccade", "DO - Export Summary", "Export - Open Summary", "Export - Summary", "DO - Export Saccades", "Export - Open Saccades", "Export - Saccades", "DO - Export Group", "Export - Open Group", "Export - Group", "Do - Export All"] ("element")
              }
            }
            n58 = for {
              tunnel: w86 -> [w90]
              tunnel: w85 -> [w89] mode=indexing
              n59 = Enqueue Element(queue=w90, element=w89) -> ()  [unwired: 2 in, 3 out]
            }
          }
        }
      }
      event Value Change {
        # "Selected plane has changed. Auto select channels?"
        n60 = event-data() -> ("NewVal"=w93:T2)  [unwired: 1 in]
        n61 = local read "bool_autoChannel"() -> (w94:bool)
        n62 = Enqueue Element(queue=w92, element=Saccade_Analyser_States."DO - Analysis") -> ()  [unwired: 2 in, 3 out]
        n63 = case shown="True" w94 {
          tunnel: w93 -> [_ w98]
          frame False {
          }
          frame True {
            n64 = call "SaccadeAnalyser - Auto Select Channels.vi"("plane"=w98) -> ("Position Response Channel"=w95:u16, "Velocity Response Channel"=w96:u16, "Stimulus Channel"=w97:u16)  [unwired: 8 in]
            n65 = local write "enum_direction"(enum16{"Positive", "Negative"}."Positive" ("enum_direction")) -> ()
            n66 = local write "ring_stimulusChannel"(w97) -> ()
            n67 = local write "ring_responseChannel"(w96) -> ()
            n68 = local write "ring_responsePosChannel"(w95) -> ()
          }
        }
      }
      event "enum_direction", "ring_responseChannel", "ring_stimulusChannel", "stim_Onset%", "gain_WinDur", "gain_WinLead", "gain_Valid%", "sac_NSampleTime", "sac_AccMin", "sac_AccMult", "sac_BiphasicCond", "bool_includePrePeak", "bool_isCoilsData": Value Change {
        # "Analysis configuration changed. Redo analysis."
        n69 = event-data() -> ()  [unwired: 1 in, 6 out]
        n70 = Enqueue Element(queue=w101, element=Saccade_Analyser_States."DO - Analysis") -> ()  [unwired: 2 in, 3 out]
      }
      event "enum_summaryType": Value Change {
        # "Summary type selection changed. Redo summary analysis."
        n71 = event-data() -> ()  [unwired: 1 in, 6 out]
        n72 = Enqueue Element(queue=w103, element=Saccade_Analyser_States."DO - Summary Analysis") -> ()  [unwired: 2 in, 3 out]
      }
      event "btn_exportSummary": Value Change {
        # "Export button pressed. Export summary data to Excel."
        n73 = event-data() -> ("NewVal"=w104:bool)  [unwired: 1 in]
        n74 = case shown="False" w104 {
          tunnel: w105 -> [_ w107]
          frame True {
          }
          frame False {
            n75 = Enqueue Element(queue=w107, element=Saccade_Analyser_States."DO - Export Summary") -> ()  [unwired: 2 in, 3 out]
          }
        }
      }
      event "btn_exportSaccades": Value Change {
        # "Export button pressed. Export saccade data to Excel."
        n76 = event-data() -> ("NewVal"=w108:bool)  [unwired: 1 in]
        n77 = case shown="False" w108 {
          tunnel: w109 -> [_ w111]
          frame True {
          }
          frame False {
            n78 = Enqueue Element(queue=w111, element=Saccade_Analyser_States."DO - Export Saccades") -> ()  [unwired: 2 in, 3 out]
          }
        }
      }
      event "btn_exportGroup": Value Change {
        # "Export button pressed. Export saccade data to Excel."
        n79 = event-data() -> ("NewVal"=w112:bool)  [unwired: 1 in]
        n80 = case shown="False" w112 {
          tunnel: w113 -> [_ w115]
          frame True {
          }
          frame False {
            n81 = Enqueue Element(queue=w115, element=Saccade_Analyser_States."DO - Export Group") -> ()  [unwired: 2 in, 3 out]
          }
        }
      }
      event "btn_exportAll": Value Change {
        # "Export button pressed. Export saccade data to Excel."
        n82 = event-data() -> ("NewVal"=w116:bool)  [unwired: 1 in]
        n83 = case shown="False" w116 {
          tunnel: w117 -> [_ w119]
          frame True {
          }
          frame False {
            n84 = Enqueue Element(queue=w119, element=Saccade_Analyser_States."Do - Export All") -> ()  [unwired: 2 in, 3 out]
          }
        }
      }
    }
  }
  n85 = while {
    tunnel: w2 -> [w129]
    shift-right: [w123] -> w7
    shift-left: "Data IN" -> [w125]
    shift-right: [w122] -> w6
    shift-left: "error in (no error)" -> [w124]
    shift-right: [w120] -> _